vi "HFRR ADV v038 new software.vi"() -> ()   [LabVIEW 2025] (continued)
        n1338 = Not(x=w1631) -> (.not. x?=w1629:bool)
        n1339 = local write "Stroke"(w1629) -> ()
        n1340 = local write "Tab Control 2"(T6."Stroke" ("Tab Control 2")) -> ()
      }
    }
    n1341 = local write "tested by"(w1358) -> ()
    n1342 = case shown="True" w1354 {
      selector: w1354 -> [_ w1634]
      frame False {
      }
      frame True {
        n1343 = Not(x=w1634) -> (.not. x?=w1632:bool)
        n1344 = local write "Humidity 2"(w1632) -> ()
        n1345 = local write "Tab Control 2"(T6."Humidity" ("Tab Control 2")) -> ()
      }
    }
    n1346 = case shown="\"Calibration\"" "Main Dashboard Buttons" {
      tunnel: [T2."HOME" ("Main Tab") T2."Test Setup" ("Main Tab") T2."Acquire" ("Main Tab") T2."Adv Scar" ("Main Tab") T2."Adv Scar Report" ("Main Tab") T2."Compare Files" ("Main Tab") T2."Calibration" ("Main Tab") T2."About" ("Main Tab") T2."Advance" ("Main Tab")] -> w1337
      frame "Home", Default {
      }
      frame "Test Setup" {
      }
      frame "Dashboard" {
      }
      frame "Imaging" {
      }
      frame "Report" {
      }
      frame "Analysis" {
      }
      frame "Calibration" {
      }
      frame "About" {
      }
      frame "Advance" {
      }
    }
    n1347 = Wait (ms)(milliseconds to wait=u32 100) -> ()  [unwired: 1 out]
    n1348 = local read "Main Tab Display"() -> (w1357:T4)
    n1349 = local write "Main Tab"(w1337) -> ()
    n1350 = case shown="\"Dashboard 3\"" w1357 {
      frame "Dashboard 1", Default {
        n1351 = property on="Reset Graph" class="Bool (strict)"("Visible"=FALSE) -> ()  [unwired: 2 in, 2 out]
      }
      frame "Dashboard 2" {
        n1352 = property on="Reset Graph" class="Bool (strict)"("Visible"=TRUE) -> ()  [unwired: 2 in, 2 out]
      }
      frame "Dashboard 3" {
        n1353 = property on="Reset Graph" class="Bool (strict)"("Visible"=TRUE) -> ()  [unwired: 2 in, 2 out]
      }
    }
    n1354 = local read "SCAR MEASURMENT"() -> (w1345:enum32{"Auto Scar", "Manual Scar"})
    n1355 = local read "Humidity"() -> (w1359:bool)
    n1356 = local read "Cap Live Image"() -> (w1342:bool)
    n1357 = local read "Sample Temperature"() -> (w1352:bool)
    n1358 = local read "Air Temp vs Humidity"() -> (w1350:bool)
    n1359 = local read "Frequency"() -> (w1351:bool)
    n1360 = case shown="True" w1359 {
      frame False {
        n1361 = local write "Humidity On Command"(TRUE ("Humidity On Command")) -> ()
        n1362 = case shown="True" "Humidity Off Command" {
          selector: "Humidity Off Command" -> [_ w1647]
          frame False {
          }
          frame True {
            n1363 = stacked-sequence {
              frame #0 {
                n1364 = Wait (ms)(milliseconds to wait=u32 500) -> ()  [unwired: 1 out]
              }
              frame #1 {
                n1365 = local read "WriteHumidity"() -> (w1650:string[])
                n1366 = Insert Into Array(array=w1650, new element="R;1" ("new element/subarray")) -> (w1649:string[])  [unwired: 1 in]
                n1367 = local write "WriteHumidity"(w1649) -> ()
              }
              frame #2 {
                n1368 = Wait (ms)(milliseconds to wait=u32 500) -> ()  [unwired: 1 out]
              }
              frame #3 {
                n1369 = local read "WriteHumidity"() -> (w1653:string[])
                n1370 = local read "EVENT LOG"() -> (w1657:string)
                n1371 = call "Event Log.vi"("Content"="Humidity Control Off" ("string"), "EVENT LOG"=w1657) -> ("EVENT LOG"=w1658:string)  [unwired: 8 in, 1 out]
                n1372 = local write "EVENT LOG"(w1658) -> ()
                n1373 = Insert Into Array(array=w1653, new element="R;1" ("new element/subarray")) -> (w1654:string[])  [unwired: 1 in]
                n1374 = local write "WriteHumidity"(w1654) -> ()
              }
            }
            n1375 = Not(x=w1647) -> (.not. x?=w1646:bool)
            n1376 = local write "Humidity Off Command"(w1646) -> ()
          }
        }
      }
      frame True {
        n1377 = local write "Humidity Off Command"(TRUE ("Humidity Off Command")) -> ()
        n1378 = case shown="True" "Humidity On Command" {
          selector: "Humidity On Command" -> [_ w1662]
          frame False {
          }
          frame True {
            n1379 = stacked-sequence {
              frame #0 {
                n1380 = local read "Set Rh"() -> (w1668:dbl)
                n1381 = local read "WriteHumidity"() -> (w1664:string[])
                n1382 = Number To Fractional String(number=w1668, precision (6)=i16 2) -> (F-format string=w1669:string)  [unwired: 2 in]
                n1383 = Concatenate Strings("M;" ("new element/subarray"), w1669) -> (w1667:string)
                n1384 = Insert Into Array(array=w1664, new element=w1667) -> (w1663:string[])  [unwired: 1 in]
                n1385 = local write "WriteHumidity"(w1663) -> ()
              }
              frame #1 {
                n1386 = Wait (ms)(milliseconds to wait=u32 500) -> ()  [unwired: 1 out]
              }
              frame #2 {
                n1387 = local read "WriteHumidity"() -> (w1672:string[])
                n1388 = local read "Set Rh"() -> (w1676:dbl)
                n1389 = Number To Fractional String(number=w1676, precision (6)=i16 2) -> (F-format string=w1677:string)  [unwired: 2 in]
                n1390 = Concatenate Strings("M;" ("new element/subarray"), w1677) -> (w1675:string)
                n1391 = Insert Into Array(array=w1672, new element=w1675) -> (w1671:string[])  [unwired: 1 in]
                n1392 = local write "WriteHumidity"(w1671) -> ()
              }
              frame #3 {
                n1393 = Wait (ms)(milliseconds to wait=u32 500) -> ()  [unwired: 1 out]
              }
              frame #4 {
                (unwired) "% RH" ("string")
                (unwired) i16 2 ("precision (6)")
                (unwired) "M;" ("new element/subarray")
                n1394 = local read "Set Rh"() -> (w1686:dbl)
                n1395 = local read "WriteHumidity"() -> (w1679:string[])
                n1396 = Number To Fractional String(number=w1686, precision (6)=i16 2) -> (F-format string=w1683:string)  [unwired: 2 in]
                n1397 = Concatenate Strings("M;" ("new element/subarray"), w1683) -> (w1687:string)
                n1398 = Concatenate Strings("Humidity Set to : " ("string"), w1683, "% RH" ("string")) -> (w1681:string)
                n1399 = Insert Into Array(array=w1679, new element=w1687) -> (w1680:string[])  [unwired: 1 in]
                n1400 = disable-structure shown="Enabled" {
                  frame Enabled {
                    n1401 = local read "EVENT LOG"() -> (w1690:string)
                    n1402 = call "Event Log.vi"("Content"="Humidity Control On", "EVENT LOG"=w1690) -> ("EVENT LOG"=w1691:string)  [unwired: 8 in, 1 out]
                    n1403 = local write "EVENT LOG"(w1691) -> ()
                  }
                  frame Disabled {
                  }
                }
                n1404 = disable-structure shown="Enabled" {
                  disable-tunnel: w1681 -> [_ _]
                  frame Enabled {
                    n1405 = local read "EVENT LOG"() -> (w1693:string)
                    n1406 = call "Event Log.vi"("Content"="Humidity Control On", "EVENT LOG"=w1693) -> ("EVENT LOG"=w1694:string)  [unwired: 8 in, 1 out]
                    n1407 = local write "EVENT LOG"(w1694) -> ()
                  }
                  frame Disabled {
                  }
                }
                n1408 = local write "WriteHumidity"(w1680) -> ()
              }
            }
            n1409 = Not(x=w1662) -> (.not. x?=w1661:bool)
            n1410 = local write "Humidity On Command"(w1661) -> ()
          }
        }
      }
    }
    n1411 = Equal?(x=w1345, y=enum32{"Auto Scar", "Manual Scar"}."Auto Scar" ("SCAR MEASURMENT")) -> (x = y?=w1341:bool)
    n1412 = local read "TEST STANDARD"() -> (w1348:T3)
    n1413 = And(x=w1342, y=w1341) -> (x .and. y?=w1343:bool)
    n1414 = case shown="True" w1343 {
      selector: w1343 -> [_ w1446]
      tunnel: errorcluster {"status"=FALSE, "code"=0, "source"=""} ("error in (no error) 3") -> [_ w1447]
      frame False {
      }
      frame True {
        n1415 = stacked-sequence {
          tunnel: w1447 -> [_ _ _ _ _ _ _ w1495]
          tunnel: w1446 -> [_ _ _ _ _ w1476 _ _]
          frame #0 {
            n1416 = call "CAMERA LIVE FEED FGV.vi"("Enum - Menu"=CAMERA_LIVE_FEED_ENUM."CAMERA MINIMIZE") -> ()  [unwired: 9 in, 2 out]
          }
          frame #1 {
            n1417 = property on="Auto Scar Check  2" class="Clust (strict)"("Visible"=TRUE) -> ()  [unwired: 2 in, 2 out]
          }
          frame #2 {
            n1418 = String To Path(string="C:\\LAB-IQ\\Image Calibrate v01.dcf") -> (path=w1452:path)
            n1419 = Open/Create/Replace File ("Open File")(file path (use dialog)=w1452) -> (refnum out=w1453:refnum<file>)  [unwired: 5 in, 2 out]
            n1420 = for {
              N: 4 -> [_]
              tunnel: w1453 -> [w1459]
              i -> [w1455]
              n1421 = Read from Text File ("Read File")(file (use dialog)=w1459) -> (text=w1460:string)  [unwired: 3 in, 3 out]
              n1422 = String Subset(string=w1460, offset (0)=6, length (rest)=10 ("length (rest)")) -> (substring=w1456:string)
              n1423 = Fract/Exp String To Number(string=w1456) -> (number=w1454:dbl)  [unwired: 3 in, 1 out]
              n1424 = case shown="0" w1455 {
                tunnel: w1454 -> [w1461 w1462 _ w1463 _]
                frame 0 {
                  "5x Gain" <- w1461
                }
                frame 1 {
                  "10x Gain" <- w1462
                }
                frame 2 {
                }
                frame 3 {
                  "100x gain" <- w1463
                }
                frame 4, Default {
                }
              }
            }
          }
          frame #3 {
            n1425 = local read "FILE 3"() -> (w1469:string)
            n1426 = call <vilib>:"Trim Whitespace.vi"("string"="C:\\LAB-IQ\\images\\") -> ("trimmed string"=w1471:string)  [unwired: 1 in]
            n1427 = String To Path(string=w1471) -> (path=w1470:path)
            n1428 = Concatenate Strings(w1469, ".png" ("string")) -> (w1468:string)
            n1429 = Build Path(base path=w1470, name or relative path=w1468) -> (appended path=w1466:path)
            "Image path" <- w1466
            n1430 = Path To String(path=w1466) -> (string=w1465:string)
            n1431 = call "CAMERA LIVE FEED FGV.vi"("Enum - Menu"=CAMERA_LIVE_FEED_ENUM."CAMERA SAVE", "Image Path"=w1465) -> ()  [unwired: 8 in, 2 out]
          }
          frame #4 {
            n1432 = One Button Dialog(message="Image saved successfully") -> ()  [unwired: 1 in, 1 out]
          }
          frame #5 {
            n1433 = local read "TEST STANDARD"() -> (w1475:T3)
            n1434 = local read "Magnification len live scar"() -> (w1487:string)
            n1435 = Not(x=w1476) -> (.not. x?=w1477:bool)
            n1436 = local write "Cap Live Image"(w1477) -> ()
            n1437 = case shown="\"ISO 12156\"" w1475 {
              tunnel: ["ASTM D6079" "ISO 12156"] -> w1474
              frame "ASTM D6079", Default {
              }
              frame "ISO 12156" {
              }
            }
            n1438 = case shown="\"5x\", Default" w1487 {
              tunnel: [w1490 w1491] -> w1486
              frame "5x", Default {
                n1439 = local read "5x Gain"() -> (w1490:dbl)
              }
              frame "10x" {
                # "5x"
                n1440 = local read "10x Gain"() -> (w1491:dbl)
              }
            }
            n1441 = local read "Image path"() -> (w1485:path)
            n1442 = local read "FILE 3"() -> (w1478:string)
            n1443 = call "EDGE DETCTION.vi"("GAIN VALUE"=w1486, "Image Path"=w1485) -> ("error out"=w1484:errorcluster, "return value"=w1483:cluster{string, string, dbl, dbl, dbl})  [unwired: 8 in]
            n1444 = Bundle By Name(cluster=T26 {"File Name"="", "Test Method"="", "Operator"="", "Fuel Description"="", "Date and time"=""} ("Main Ref"), "File Name"=w1478, "Test Method"=w1474) -> (w1479:T26)
            n1445 = call "duf file read.vi"("error in (no error)"=w1484, "Main Ref"=w1479) -> ("error out"=w1482:errorcluster, "Main Ref 2"=w1480:T26)  [unwired: 8 in]
            n1446 = call "EDGE DETECTION REPORT.vi"("error in (no error)"=w1482, "return value 2"=w1483, "Main Ref"=w1480) -> ()  [unwired: 8 in, 1 out]
          }
          frame #6 {
            n1447 = property on="Auto Scar Check  2" class="Clust (strict)"("Visible"=FALSE) -> ()  [unwired: 2 in, 2 out]
          }
          frame #7 {
            n1448 = call "CAMERA LIVE FEED FGV.vi"("Enum - Menu"=CAMERA_LIVE_FEED_ENUM."CAMERA MINIMIZE", "error in (no error)"=w1495) -> ()  [unwired: 8 in, 2 out]
            n1449 = local write "Main Dashboard Buttons"(T1."Home" ("Main Dashboard Buttons")) -> ()
            n1450 = local write "Main Tab"(T2."HOME" ("Main Tab")) -> ()
          }
        }
      }
    }
    n1451 = local read "Heater Button"() -> (w1349:bool)
    n1452 = case shown="True" w1351 {
      selector: w1351 -> [_ w1625]
      frame False {
      }
      frame True {
        n1453 = Not(x=w1625) -> (.not. x?=w1623:bool)
        n1454 = local write "Frequency"(w1623) -> ()
        n1455 = local write "Tab Control 2"(T6."Frequency" ("Tab Control 2")) -> ()
      }
    }
    n1456 = case shown="True" w1350 {
      selector: w1350 -> [_ w1622]
      frame False {
      }
      frame True {
        n1457 = Not(x=w1622) -> (.not. x?=w1620:bool)
        n1458 = local write "Air Temp vs Humidity"(w1620) -> ()
        n1459 = local write "Tab Control 2"(T6."Air Temp vs Rh" ("Tab Control 2")) -> ()
      }
    }
    n1460 = case shown="True" w1352 {
      selector: w1352 -> [_ w1628]
      frame False {
      }
      frame True {
        n1461 = Not(x=w1628) -> (.not. x?=w1626:bool)
        n1462 = local write "Sample Temperature"(w1626) -> ()
        n1463 = local write "Tab Control 2"(T6."Sample Temperature" ("Tab Control 2")) -> ()
      }
    }
    n1464 = case shown="\"Custom\"" w1348 {
      frame "ASTM D6079", Default {
        w1601 = "ASTM D6079 TEST CONDITIONS" ("Standard 2")
        n1465 = local write "Standard 2"(w1601) -> ()
        n1466 = local write "Standard"(w1601) -> ()
      }
      frame "ISO 12156" {
        w1602 = "ISO 12156 TEST CONDITIONS" ("Standard 2")
        n1467 = local write "Standard 2"(w1602) -> ()
        n1468 = local write "Standard"(w1602) -> ()
      }
      frame "CEC F-096-A-06" {
        w1603 = "CEC F-096-A-06 TEST CONDITIONS" ("Standard 2")
        n1469 = local write "Standard 2"(w1603) -> ()
        n1470 = local write "Standard"(w1603) -> ()
      }
      frame "Custom" {
        w1604 = "CUSTOM TEST CONDITIONS" ("Standard 2")
        n1471 = local write "Standard 2"(w1604) -> ()
        n1472 = local write "Standard"(w1604) -> ()
      }
    }
    n1473 = case shown="True" w1349 {
      frame False {
        n1474 = local write "Temperature On Command"(TRUE ("Temperature On Command")) -> ()
        n1475 = case shown="True" "Temperature Off Command" {
          selector: "Temperature Off Command" -> [_ w1608]
          frame False {
          }
          frame True {
            n1476 = Not(x=w1608) -> (.not. x?=w1607:bool)
            n1477 = local read "EVENT LOG"() -> (w1611:string)
            n1478 = local write "Temperature Off Command"(w1607) -> ()
            n1479 = call "Event Log.vi"("Content"="Heater Off", "EVENT LOG"=w1611) -> ("EVENT LOG"=w1610:string)  [unwired: 8 in, 1 out]
            n1480 = local write "EVENT LOG"(w1610) -> ()
          }
        }
      }
      frame True {
        n1481 = local write "Temperature Off Command"(TRUE ("Temperature Off Command")) -> ()
        n1482 = case shown="True" "Temperature On Command" {
          selector: "Temperature On Command" -> [_ w1615]
          frame False {
          }
          frame True {
            n1483 = Not(x=w1615) -> (.not. x?=w1614:bool)
            n1484 = local write "Temperature On Command"(w1614) -> ()
            n1485 = disable-structure shown="Enabled" {
              disable-tunnel: "Heater On" -> [w1617 _]
              frame Enabled {
                n1486 = local read "EVENT LOG"() -> (w1618:string)
                n1487 = call "Event Log.vi"("Content"=w1617, "EVENT LOG"=w1618) -> ("EVENT LOG"=w1619:string)  [unwired: 8 in, 1 out]
                n1488 = local write "EVENT LOG"(w1619) -> ()
              }
              frame Disabled {
              }
            }
          }
        }
      }
    }
    n1489 = local read "Main Tab"() -> (w1340:T2)
    n1490 = case shown="\"About\"" w1340 {
      frame "HOME", Default {
        w1382 = T19."Enabled" ("Disabled")
        n1491 = local read "Service Password enable"() -> (w1384:bool)
        n1492 = property on="Imaging" class="Bool (strict)"("DisabledEnum"=w1382) -> ()  [unwired: 2 in, 2 out]
        n1493 = property on="Dashboard" class="Bool (strict)"("DisabledEnum"=w1382) -> ()  [unwired: 2 in, 2 out]
        n1494 = property on="Test Setup" class="Bool (strict)"("DisabledEnum"=w1382) -> ()  [unwired: 2 in, 2 out]
        n1495 = property on="Analysis" class="Bool (strict)"("DisabledEnum"=w1382) -> ()  [unwired: 2 in, 2 out]
        n1496 = property on="Home" class="Bool (strict)"("DisabledEnum"=w1382) -> ()  [unwired: 2 in, 2 out]
        n1497 = property on="Report" class="Bool (strict)"("DisabledEnum"=w1382) -> ()  [unwired: 2 in, 2 out]
        n1498 = property on="Main Dashboard Buttons" class="RadioBtnsControl (strict)"("DisabledEnum"=w1382) -> ()  [unwired: 2 in, 2 out]
        n1499 = property on="Calibration" class="Bool (strict)"("DisabledEnum"=w1382) -> ()  [unwired: 2 in, 2 out]
        n1500 = case shown="True" w1384 {
          tunnel: [T19."Disabled" ("Disabled") T19."Enabled" ("Disabled")] -> w1383
          frame False {
          }
          frame True {
          }
        }
        n1501 = property on="About" class="Bool (strict)"("DisabledEnum"=w1383) -> ()  [unwired: 2 in, 2 out]
      }
      frame "Test Setup" {
        w1389 = T19."Enabled" ("Disabled")
        n1502 = local read "Service Password enable"() -> (w1388:bool)
        n1503 = property on="Dashboard" class="Bool (strict)"("DisabledEnum"=T19."Disabled" ("Disabled")) -> ()  [unwired: 2 in, 2 out]
        n1504 = property on="Imaging" class="Bool (strict)"("DisabledEnum"=w1389) -> ()  [unwired: 2 in, 2 out]
        n1505 = property on="Analysis" class="Bool (strict)"("DisabledEnum"=w1389) -> ()  [unwired: 2 in, 2 out]
        n1506 = property on="Home" class="Bool (strict)"("DisabledEnum"=w1389) -> ()  [unwired: 2 in, 2 out]
        n1507 = property on="Report" class="Bool (strict)"("DisabledEnum"=w1389) -> ()  [unwired: 2 in, 2 out]
        n1508 = property on="Test Setup" class="Bool (strict)"("DisabledEnum"=w1389) -> ()  [unwired: 2 in, 2 out]
        n1509 = case shown="True" w1388 {
          tunnel: [T19."Disabled" ("Disabled") T19."Enabled" ("Disabled")] -> w1387
          frame False {
          }
          frame True {
          }
        }
        n1510 = property on="About" class="Bool (strict)"("DisabledEnum"=w1387) -> ()  [unwired: 2 in, 2 out]
      }
      frame "Adv Scar" {
        w1396 = T19."Enabled" ("Disabled")
        n1511 = property on="Dashboard" class="Bool (strict)"("DisabledEnum"=T19."Disabled" ("Disabled")) -> ()  [unwired: 2 in, 2 out]
        n1512 = property on="Imaging" class="Bool (strict)"("DisabledEnum"=w1396) -> ()  [unwired: 2 in, 2 out]
        n1513 = property on="Analysis" class="Bool (strict)"("DisabledEnum"=w1396) -> ()  [unwired: 2 in, 2 out]
        n1514 = property on="Home" class="Bool (strict)"("DisabledEnum"=w1396) -> ()  [unwired: 2 in, 2 out]
        n1515 = property on="Report" class="Bool (strict)"("DisabledEnum"=w1396) -> ()  [unwired: 2 in, 2 out]
        n1516 = property on="Test Setup" class="Bool (strict)"("DisabledEnum"=w1396) -> ()  [unwired: 2 in, 2 out]
        n1517 = local read "Service Password enable"() -> (w1394:bool)
        n1518 = case shown="True" w1394 {
          tunnel: [T19."Disabled" ("Disabled") T19."Enabled" ("Disabled")] -> w1393
          frame False {
          }
          frame True {
          }
        }
        n1519 = property on="About" class="Bool (strict)"("DisabledEnum"=w1393) -> ()  [unwired: 2 in, 2 out]
      }
      frame "Calibration" {
        w1399 = T19."Enabled" ("Disabled")
        n1520 = property on="Dashboard" class="Bool (strict)"("DisabledEnum"=T19."Disabled" ("Disabled")) -> ()  [unwired: 2 in, 2 out]
        n1521 = property on="Imaging" class="Bool (strict)"("DisabledEnum"=w1399) -> ()  [unwired: 2 in, 2 out]
        n1522 = property on="Analysis" class="Bool (strict)"("DisabledEnum"=w1399) -> ()  [unwired: 2 in, 2 out]
        n1523 = property on="Home" class="Bool (strict)"("DisabledEnum"=w1399) -> ()  [unwired: 2 in, 2 out]
        n1524 = property on="Report" class="Bool (strict)"("DisabledEnum"=w1399) -> ()  [unwired: 2 in, 2 out]
        n1525 = property on="Test Setup" class="Bool (strict)"("DisabledEnum"=w1399) -> ()  [unwired: 2 in, 2 out]
        n1526 = local read "Service Password enable"() -> (w1401:bool)
        n1527 = property on="Calibration" class="Bool (strict)"("DisabledEnum"=w1399) -> ()  [unwired: 2 in, 2 out]
        n1528 = case shown="True" w1401 {
          tunnel: [T19."Disabled" ("Disabled") T19."Enabled" ("Disabled")] -> w1400
          frame False {
          }
          frame True {
          }
        }
        n1529 = property on="About" class="Bool (strict)"("DisabledEnum"=w1400) -> ()  [unwired: 2 in, 2 out]
      }
      frame "Adv Scar Report" {
        w1407 = T19."Enabled" ("Disabled")
        n1530 = property on="Dashboard" class="Bool (strict)"("DisabledEnum"=T19."Disabled" ("Disabled")) -> ()  [unwired: 2 in, 2 out]
        n1531 = property on="Imaging" class="Bool (strict)"("DisabledEnum"=w1407) -> ()  [unwired: 2 in, 2 out]
        n1532 = property on="Analysis" class="Bool (strict)"("DisabledEnum"=w1407) -> ()  [unwired: 2 in, 2 out]
        n1533 = property on="Home" class="Bool (strict)"("DisabledEnum"=w1407) -> ()  [unwired: 2 in, 2 out]
        n1534 = property on="Report" class="Bool (strict)"("DisabledEnum"=w1407) -> ()  [unwired: 2 in, 2 out]
        n1535 = property on="Test Setup" class="Bool (strict)"("DisabledEnum"=w1407) -> ()  [unwired: 2 in, 2 out]
        n1536 = local read "Service Password enable"() -> (w1406:bool)
        n1537 = case shown="True" w1406 {
          tunnel: [T19."Disabled" ("Disabled") T19."Enabled" ("Disabled")] -> w1405
          frame False {
          }
          frame True {
          }
        }
        n1538 = property on="About" class="Bool (strict)"("DisabledEnum"=w1405) -> ()  [unwired: 2 in, 2 out]
      }
      frame "Compare Files" {
        w1413 = T19."Enabled" ("Disabled")
        n1539 = local read "Service Password enable"() -> (w1412:bool)
        n1540 = property on="Dashboard" class="Bool (strict)"("DisabledEnum"=T19."Disabled" ("Disabled")) -> ()  [unwired: 2 in, 2 out]
        n1541 = property on="Imaging" class="Bool (strict)"("DisabledEnum"=w1413) -> ()  [unwired: 2 in, 2 out]
        n1542 = property on="Analysis" class="Bool (strict)"("DisabledEnum"=w1413) -> ()  [unwired: 2 in, 2 out]
        n1543 = property on="Home" class="Bool (strict)"("DisabledEnum"=w1413) -> ()  [unwired: 2 in, 2 out]
        n1544 = property on="Report" class="Bool (strict)"("DisabledEnum"=w1413) -> ()  [unwired: 2 in, 2 out]
        n1545 = property on="Test Setup" class="Bool (strict)"("DisabledEnum"=w1413) -> ()  [unwired: 2 in, 2 out]
        n1546 = case shown="True" w1412 {
          tunnel: [T19."Disabled" ("Disabled") T19."Enabled" ("Disabled")] -> w1411
          frame False {
          }
          frame True {
          }
        }
        n1547 = property on="About" class="Bool (strict)"("DisabledEnum"=w1411) -> ()  [unwired: 2 in, 2 out]
      }
      frame "Acquire" {
        n1548 = local read "Service Password enable"() -> (w1418:bool)
        n1549 = property on="Test Setup" class="Bool (strict)"("DisabledEnum"=T19."Disabled" ("Disabled")) -> ()  [unwired: 2 in, 2 out]
        n1550 = local read "Auto Start Test"() -> (w1420:bool)
        n1551 = local read "RUN"() -> (w1422:bool)
        n1552 = case shown="True" w1418 {
          tunnel: [T19."Disabled" ("Disabled") T19."Enabled" ("Disabled")] -> w1419
          frame False {
          }
          frame True {
          }
        }
        n1553 = Or(x=w1422, y=w1420) -> (x .or. y?=w1421:bool)
        n1554 = case shown="True" w1421 {
          tunnel: [T19."Enabled" ("Disabled") T19."Disabled" ("Disabled")] -> w1417
          frame False {
          }
          frame True {
          }
        }
        n1555 = property on="About" class="Bool (strict)"("DisabledEnum"=w1419) -> ()  [unwired: 2 in, 2 out]
        n1556 = property on="Imaging" class="Bool (strict)"("DisabledEnum"=w1417) -> ()  [unwired: 2 in, 2 out]
        n1557 = property on="Dashboard" class="Bool (strict)"("DisabledEnum"=w1417) -> ()  [unwired: 2 in, 2 out]
        n1558 = property on="Analysis" class="Bool (strict)"("DisabledEnum"=w1417) -> ()  [unwired: 2 in, 2 out]
        n1559 = property on="Home" class="Bool (strict)"("DisabledEnum"=w1417) -> ()  [unwired: 2 in, 2 out]
        n1560 = property on="Report" class="Bool (strict)"("DisabledEnum"=w1417) -> ()  [unwired: 2 in, 2 out]
        n1561 = property on="Calibration" class="Bool (strict)"("DisabledEnum"=w1417) -> ()  [unwired: 2 in, 2 out]
      }
      frame "About" {
        n1562 = local read "FILE"() -> (w1436:string)
        n1563 = local read "TEST FILE NAM,E SAVED"() -> (w1429:bool)
        n1564 = call <vilib>:"Trim Whitespace.vi"("string"=w1436) -> ("trimmed string"=w1435:string)  [unwired: 1 in]
        n1565 = local read "Auto Start Test"() -> (w1439:bool)
        n1566 = String Length(string=w1435) -> (length=w1434:i32)
        n1567 = Greater?(x=w1434, y=1) -> (0:w1431:bool)
        n1568 = And(x=w1431, y=w1429) -> (x .and. y?=w1430:bool)
        n1569 = local read "RUN"() -> (w1441:bool)
        n1570 = case shown="True" w1430 {
          tunnel: [T19."Disabled" ("Disabled") T19."Enabled" ("Disabled")] -> w1432
          frame False {
          }
          frame True {
          }
        }
        n1571 = Or(x=w1441, y=w1439) -> (x .or. y?=w1440:bool)
        n1572 = property on="About" class="Bool (strict)"("DisabledEnum"=T19."Enabled" ("Disabled")) -> ()  [unwired: 2 in, 2 out]
        n1573 = case shown="False" w1440 {
          tunnel: [T19."Enabled" ("Disabled") T19."Disabled" ("Disabled")] -> w1438
          frame False {
          }
          frame True {
          }
        }
        n1574 = property on="Dashboard" class="Bool (strict)"("DisabledEnum"=w1432) -> ()  [unwired: 2 in, 2 out]
        n1575 = property on="Test Setup" class="Bool (strict)"("DisabledEnum"=T19."Disabled" ("Disabled")) -> ()  [unwired: 2 in, 2 out]
        n1576 = property on="Imaging" class="Bool (strict)"("DisabledEnum"=w1438) -> ()  [unwired: 2 in, 2 out]
        n1577 = property on="Analysis" class="Bool (strict)"("DisabledEnum"=w1438) -> ()  [unwired: 2 in, 2 out]
        n1578 = property on="Home" class="Bool (strict)"("DisabledEnum"=w1438) -> ()  [unwired: 2 in, 2 out]
        n1579 = property on="Report" class="Bool (strict)"("DisabledEnum"=w1438) -> ()  [unwired: 2 in, 2 out]
      }
    }
    n1580 = local read "Quit"() -> (w1366:bool)
    "Single" <- "Single - Graph"
  }
  n1581 = disable-structure shown="Disabled" {
    disable-tunnel: [w1719 _] -> w42
    disable-tunnel: _ -> [w1718 _]
    frame Disabled {
      n1582 = while {
        tunnel: w1718 -> [_]
        tunnel: [w1720] -> w1719
        tunnel: [w1721] -> _
        i -> [w1721]
        stop <- w1720 stop-if-true
        w1737 = u16 10 items=["1.0"=10, "1.5"=15, "2.0"=20] ("stop bits (10: 1 bit)")
        n1583 = Wait (ms)(milliseconds to wait=u32 10) -> ()  [unwired: 1 out]
        n1584 = call-poly "VISA Configure Serial Port"("VISA resource name"=refnum<visa-resource-name> "ASRL1::INSTR" ("COM PORT"), "timeout (10sec)"=u32 10, "baud rate (9600)"=u32 57600, "data bits (8)"=u16 8, "stop bits (10: 1 bit)"=w1737) -> ("VISA resource name out"=w1723:refnum<visa-resource-name>, "error out"=w1732:errorcluster)  [unwired: 9 in]
        n1585 = VISA Read(VISA resource name=w1723, byte count=u32 2 ("byte count (0)")) -> (read buffer=w1731:string)  [unwired: 1 in, 3 out]
        n1586 = String Subset(string=w1731, offset (0)=0, length (rest)=2 ("length (rest)")) -> (substring=w1730:string)
        n1587 = Match Pattern(string=w1730, regular expression="<>") -> (offset past match=w1727:i32)  [unwired: 1 in, 3 out]
        n1588 = Greater Or Equal?(x=w1727, y=0) -> (x >= y?=w1722:bool)
        n1589 = case shown="True" w1722 {
          tunnel: w1723 -> [_ w1741]
          tunnel: w1732 -> [_ w1740]
          frame False {
          }
          frame True {
            n1590 = VISA Read(VISA resource name=w1741, byte count=u32 32 ("byte count (0)"), error in (no error)=w1740) -> (read buffer=w1739:string)  [unwired: 3 out]
            n1591 = String Subset(string=w1739, offset (0)=0, length (rest)=8 ("length (rest)")) -> (substring=w1743:string)
            n1592 = String Subset(string=w1739, offset (0)=8, length (rest)=8 ("length (rest)")) -> (substring=w1744:string)
            n1593 = Decimal String To Number(string=w1744) -> (number=w1751:i32)  [unwired: 2 in, 1 out]
            n1594 = Decimal String To Number(string=w1743) -> (number=w1747:i32)  [unwired: 2 in, 1 out]
            n1595 = Divide(x=w1751, y=10000) -> ()  [unwired: 1 out]
            n1596 = Divide(x=w1747, y=1000000) -> ()  [unwired: 1 out]
          }
        }
        n1597 = local read "Quit"() -> (w1720:bool)
      }
    }
    frame Enabled {
    }
  }
  n1598 = Tick Count (ms)() -> (millisecond timer value=w4:u32)
  n1599 = while {
    shift-right: [w1797] -> _
    shift-left: w6 -> [w1801]
    shift-right: [w1796] -> _
    shift-left: w5 -> [w1800]
    shift-right: [w1795] -> _
    shift-left: w6 -> [w1799]
    shift-right: [w1794] -> _
    shift-left: w5 -> [w1798]
    shift-right: [w1792] -> _
    shift-left: w4 -> [w1793]
    shift-right: [w1789] -> _
    shift-left: w3 -> [w1790]
    shift-right: [w1788] -> _
    shift-left: w3 -> [w1791]
    shift-right: [w1781] -> _
    shift-left: w3 -> [w1787]
    shift-right: [w1780] -> _
    shift-left: w3 -> [w1786]
    shift-right: [w1779] -> _
    shift-left: w3 -> [w1785]
    shift-right: [w1778] -> _
    shift-left: w3 -> [w1784]
    shift-right: [w1777] -> _
    shift-left: w3 -> [w1783]
    shift-right: [w1776] -> _
    shift-left: w3 -> [w1782]
    shift-right: [w1775] -> _
    shift-left: w3 -> [w1769]
    shift-right: [w1774] -> _
    shift-left: w3 -> [w1768]
    shift-right: [w1773] -> _
    shift-left: w3 -> [w1767]
    shift-right: [w1772] -> _
    shift-left: w3 -> [w1766]
    shift-right: [w1771] -> _
    shift-left: w3 -> [w1765]
    shift-right: [w1770] -> _
    shift-left: w3 -> [w1764]
    shift-right: [w1755] -> _
    shift-left: w3 -> [w1758]
    shift-right: [w1754] -> _
    shift-left: w3 -> [w1757]
    shift-right: [w1753] -> _
    shift-left: w3 -> [w1756]
    stop <- w1803 stop-if-true
    n1600 = local read "Read UNO"() -> (w1762:string)
    n1601 = local read "Error  2"() -> (w1802:errorcluster)
    n1602 = String Length(string=w1762) -> (length=w1761:i32)
    n1603 = call <vilib>:"Trim Whitespace.vi"("string"=w1762) -> ("trimmed string"=w1763:string)  [unwired: 1 in]
    n1604 = Greater Or Equal?(x=w1761, y=23) -> (x >= y?=w1759:bool)
    n1605 = case shown="No Error" w1802 {
      tunnel: w1801 -> [w1849 w1945]
      tunnel: w1800 -> [w1848 w1944]
      tunnel: w1799 -> [w1847 w1943]
      tunnel: w1798 -> [w1846 w1942]
      tunnel: [w1845 w1945] -> w1797
      tunnel: [w1844 w1944] -> w1796
      tunnel: [w1843 w1943] -> w1795
      tunnel: [w1842 w1942] -> w1794
      tunnel: w1793 -> [w1841 w1941]
      tunnel: [w1840 w1941] -> w1792
      tunnel: w1790 -> [w1839 w1940]
      tunnel: w1791 -> [w1838 w1939]
      tunnel: [w1837 w1940] -> w1789
      tunnel: [w1836 w1939] -> w1788
      tunnel: w1787 -> [w1835 w1938]
      tunnel: w1786 -> [w1834 w1937]
      tunnel: w1785 -> [w1833 w1936]
      tunnel: w1784 -> [w1832 w1935]
      tunnel: w1783 -> [w1831 w1934]
      tunnel: w1782 -> [w1830 w1933]
      tunnel: [w1829 w1938] -> w1781
      tunnel: [w1828 w1937] -> w1780
      tunnel: [w1827 w1936] -> w1779
      tunnel: [w1826 w1935] -> w1778
      tunnel: [w1825 w1934] -> w1777
      tunnel: [w1824 w1933] -> w1776
      tunnel: w1769 -> [w1823 w1932]
      tunnel: [w1822 w1932] -> w1775
      tunnel: [w1821 w1928] -> w1774
      tunnel: [w1820 w1927] -> w1773
      tunnel: [w1819 w1931] -> w1772
      tunnel: [w1818 w1930] -> w1771
      tunnel: [w1817 w1929] -> w1770
      tunnel: w1768 -> [w1816 w1931]
      tunnel: w1767 -> [w1815 w1930]
      tunnel: w1766 -> [w1814 w1929]
      tunnel: w1765 -> [w1813 w1928]
      tunnel: w1764 -> [w1812 w1927]
      tunnel: w1763 -> [w1811 _]
      tunnel: w1759 -> [w1810 _]
      tunnel: w1758 -> [w1809 w1926]
      tunnel: w1757 -> [w1808 w1925]
      tunnel: w1756 -> [w1807 w1924]
      tunnel: [w1806 w1926] -> w1755
      tunnel: [w1805 w1925] -> w1754
      tunnel: [w1804 w1924] -> w1753
      frame No Error {
        n1606 = case shown="True" w1810 {
          tunnel: w1849 -> [w1865 w1917]
          tunnel: w1848 -> [w1864 w1916]
          tunnel: w1847 -> [w1863 w1915]
          tunnel: w1846 -> [w1862 w1914]
          tunnel: [w1865 w1913] -> w1845
          tunnel: [w1864 w1912] -> w1844
          tunnel: [w1863 w1911] -> w1843
          tunnel: [w1862 w1910] -> w1842
          tunnel: w1841 -> [w1861 w1908]
          tunnel: [w1861 w1907] -> w1840
          tunnel: w1839 -> [w1860 w1906]
          tunnel: w1838 -> [w1859 w1905]
          tunnel: [w1860 w1904] -> w1837
          tunnel: [w1859 w1903] -> w1836
          tunnel: w1835 -> [w1858 w1902]
          tunnel: w1834 -> [w1857 w1901]
          tunnel: w1833 -> [w1856 w1900]
          tunnel: w1832 -> [w1855 w1899]
          tunnel: w1831 -> [w1854 w1898]
          tunnel: w1830 -> [w1853 w1897]
          tunnel: [w1858 w1896] -> w1829
          tunnel: [w1857 w1895] -> w1828
          tunnel: [w1856 w1894] -> w1827
          tunnel: [w1855 w1893] -> w1826
          tunnel: [w1854 w1892] -> w1825
          tunnel: [w1853 w1891] -> w1824
          tunnel: w1823 -> [w1871 w1890]
          tunnel: [w1871 w1889] -> w1822
          tunnel: [w1868 w1888] -> w1821
          tunnel: [w1867 w1887] -> w1820
          tunnel: [w1870 w1886] -> w1819
          tunnel: [w1866 w1885] -> w1818
          tunnel: [w1869 w1884] -> w1817
          tunnel: w1816 -> [w1870 w1883]
          tunnel: w1815 -> [w1869 w1882]
          tunnel: w1814 -> [w1868 w1881]
          tunnel: w1813 -> [w1867 w1880]
          tunnel: w1812 -> [w1866 w1879]
          tunnel: w1811 -> [_ w1878]
          tunnel: w1809 -> [w1852 w1877]
          tunnel: w1808 -> [w1851 w1876]
          tunnel: w1807 -> [w1850 w1875]
          tunnel: [w1852 w1874] -> w1806
          tunnel: [w1851 w1873] -> w1805
          tunnel: [w1850 w1872] -> w1804
          frame False {
          }
          frame True {
            n1607 = Tick Count (ms)() -> (millisecond timer value=w1909:u32)
            n1608 = String To Byte Array(string=w1878) -> (unsigned byte array=w1922:u8[])
            n1609 = Array Size(array=w1922) -> (size(s)=w1921:i32)
            n1610 = formula code="// --- INTERNAL VARIABLE DECLARATIONS ---\nint i = 0;\nint k = 0;\nint start_idx = -1;\nint end_idx = -1;\nint phase = 0;\nint sign0 = 1;\nint sign1 = 1;\nint ch0_val = 0;   \nint ch1_val = 0;   \nfloat ch0_raw = 0.0;\nfloat ch1_raw = 0.0;\nfloat temp0 = 0.0;\nfloat temp1 = 0.0;\nfloat ch0_clean = 0.0;\nfloat ch1_clean = 0.0;\n\nint valid_samples = 0; // FIX: Track if we actually parsed new data this window\nfloat max_allowed_bits = 8388607.0; // FIX: Change this to match your ADC max value\n\n// Temporal intermediate variables for calculation smoothing\nfloat raw_p2p_v = 0.0;\nfloat raw_friction = 0.0;\nfloat raw_cof = 0.0;\n\n// Temporal intermediate variables for Piezo voltage translations\nfloat piezo_min_v = 0.0;\nfloat piezo_max_v = 0.0;\n\n// Initialize output variables to current shift register states right away\nout_LVDT_Min_V = in_LVDT_Min_V;\nout_LVDT_Max_V = in_LVDT_Max_V;\nout_LVDT_P2P_V = in_LVDT_P2P_V;\nout_Piezo_P2P = in_Piezo_P2P;\nout_Friction_N = in_Friction_N;\nout_COF = in_COF;\nwindow_ready = 0;\n\n// --- STEP 1: PARSE EVERY STRING IN THE BYTE ARRAY ---\nif (array_size > 2) {\n    for (i = 0; i < array_size - 1; i++) {\n        if (raw_bytes[i] == 42) { // '*' character detected\n            start_idx = i;\n        }\n        \n        // Match standard delimiter sequence \";&\" or end window character\n        if (raw_bytes[i] == 59 && raw_bytes[i+1] == 38 && start_idx != -1) { \n            end_idx = i;\n            ch0_val = 0;\n            ch1_val = 0;\n            sign0 = 1;\n            sign1 = 1;\n            phase = 0; \n\n            for (k = start_idx + 1; k < end_idx; k++) {\n                if (raw_bytes[k] == 45) { // '-' sign\n                    if (phase == 0) sign0 = -1;\n                    else sign1 = -1;\n                }\n                else if (raw_bytes[k] == 43) { // '+' sign\n                    if (phase == 0) sign0 = 1;\n                    else sign1 = 1;\n                }\n                else if (raw_bytes[k] == 59) { // ';' delimiter\n                    phase = 1; \n                }\n                else if (raw_bytes[k] >= 48 && raw_bytes[k] <= 57) { // Numeric ASCII digits\n                    if (phase == 0) {\n                        ch0_val = (ch0_val * 10) + (raw_bytes[k] - 48);\n                    } else {\n                        ch1_val = (ch1_val * 10) + (raw_bytes[k] - 48);\n                    }\n                }\n            }\n\n            // Implicit type conversion\n            ch0_raw = ch0_val * sign0 * 1.0;\n            ch1_raw = ch1_val * sign1 * 1.0;\n\n            // FIX: Sanity check / Hard-clamping to catch sudden massive ASCII noise spikes\n            if (ch0_raw > max_allowed_bits)  ch0_raw = max_allowed_bits;\n            if (ch0_raw < -max_allowed_bits) ch0_raw = -max_allowed_bits;\n            if (ch1_raw > max_allowed_bits)  ch1_raw = max_allowed_bits;\n            if (ch1_raw < -max_allowed_bits) ch1_raw = -max_allowed_bits;\n\n            // --- STEP 2: 3-SAMPLE MEDIAN FILTER ---\n            m0_2 = m0_1; m0_1 = m0_0; m0_0 = ch0_raw;\n            float s0_0 = m0_0; float s0_1 = m0_1; float s0_2 = m0_2;\n            if (s0_0 > s0_1) { temp0 = s0_0; s0_0 = s0_1; s0_1 = temp0; }\n            if (s0_1 > s0_2) { temp0 = s0_1; s0_1 = s0_2; s0_2 = temp0; }\n            if (s0_0 > s0_1) { temp0 = s0_0; s0_0 = s0_1; s0_1 = temp0; }\n            ch0_clean = s0_1;\n\n            m1_2 = m1_1; m1_1 = m1_0; m1_0 = ch1_raw;\n            float s1_0 = m1_0; float s1_1 = m1_1; float s1_2 = m1_2;\n            if (s1_0 > s1_1) { temp1 = s1_0; s1_0 = s1_1; s1_1 = temp1; }\n            if (s1_1 > s1_2) { temp1 = s1_1; s1_1 = s1_2; s1_2 = temp1; }\n            if (s1_0 > s1_1) { temp1 = s1_0; s1_0 = s1_1; s1_1 = temp1; }\n            ch1_clean = s1_1;\n\n            // --- STEP 3: EXPONENTIAL FILTER (STREAM LEVEL) ---\n            if (ch0_filt == 0.0) ch0_filt = ch0_clean;\n            if (ch1_filt == 0.0) ch1_filt = ch1_clean;\n\n            ch0_filt = ch0_filt + (ch0_clean - ch0_filt) * 0.125;\n            ch1_filt = ch1_filt + (ch1_clean - ch1_filt) * 0.125;\n\n            // --- STEP 4: MIN/MAX WINDOW CONTINUOUS ACCUMULATION ---\n            if (ch0_filt > max_ch0) max_ch0 = ch0_filt;\n            if (ch0_filt < min_ch0) min_ch0 = ch0_filt;\n            if (ch1_filt > max_ch1) max_ch1 = ch1_filt;\n            if (ch1_filt < min_ch1) min_ch1 = ch1_filt;\n\n            valid_samples++; // FIX: Successfully parsed and accumulated a clean point\n            start_idx = -1; \n        }\n    }\n}\n\n// --- STEP 5: WINDOW EVALUATION ENGINE ---\n// FIX: Condition updated to verify that valid samples exist for both channels\nif (((current_time_ms - start_time_ms) >= 50) && (valid_samples > 0) && (min_ch0 < 9000000.0) && (min_ch1 < 9000000.0)) {\n    window_ready = 1;\n\n    // Linear Bit-to-Voltage Transformations (LVDT - Channel 0)\n    out_LVDT_Min_V = (min_ch0 * VREF) / 8388607.0;\n    out_LVDT_Max_V = (max_ch0 * VREF) / 8388607.0;\n    raw_p2p_v = out_LVDT_Max_V - out_LVDT_Min_V;\n\n    // Linear Bit-to-Voltage Transformations (Piezo - Channel 1)\n    piezo_min_v = (min_ch1 * VREF) / 8388607.0;\n    piezo_max_v = (max_ch1 * VREF) / 8388607.0;\n    \n    // Assign Peak-to-Peak Voltage directly to output indicator (Matches Python logic)\n    out_Piezo_P2P = piezo_max_v - piezo_min_v;\n    \n    // Force scaling calculations using Voltage delta * Newtons/Volt Factor\n    raw_friction = out_Piezo_P2P * PIEZO_CAL_FACTOR + 0.44528;\n    raw_cof = raw_friction / NORMAL_FORCE;\n\n    // --- STEP 6: OUTPUT METRIC SMOOTHING (Low-Pass Filter Alpha = 0.05) ---\n    // Seed initial historical metrics if first loop iteration\n    if (hist_LVDT_P2P == 0.0) hist_LVDT_P2P = raw_p2p_v;\n    if (hist_Friction == 0.0) hist_Friction = raw_friction;\n    if (hist_COF == 0.0)      hist_COF = raw_cof;\n\n    // Apply exponential output dampening\n    hist_LVDT_P2P = hist_LVDT_P2P + (raw_p2p_v - hist_LVDT_P2P) * 0.05;\n    hist_Friction = hist_Friction + (raw_friction - hist_Friction) * 0.05; // Note: Can drop to 0.02 for more aggressive damping\n    hist_COF      = hist_COF + (raw_cof - hist_COF) * 0.05;\n\n    // Direct smoothed parameters out to UI Indicators\n    out_LVDT_P2P_V = hist_LVDT_P2P;\n    out_Friction_N = hist_Friction;\n    out_COF        = hist_COF;\n\n    // Reset tracking targets to extreme boundaries safely\n    min_ch0 = 9999999.0;\n    max_ch0 = -9999999.0;\n    min_ch1 = 9999999.0;\n    max_ch1 = -9999999.0;\n\n    valid_samples = 0; // FIX: Reset counter for next time frame\n    start_time_ms = current_time_ms;\n}"("raw_bytes"=w1922, "array_size"=w1921, "VREF"="VREF", "PIEZO_CAL_FACTOR"="PIEZO_CAL_FACTOR", "NORMAL_FORCE"="NORMAL_FORCE", "min_ch0"=w1917, "max_ch0"=w1916, "min_ch1"=w1915, "max_ch1"=w1914, "current_time_ms"=w1909, "start_time_ms"=w1908, "ch0_filt"=w1906, "ch1_filt"=w1905, "m0_0"=w1902, "m0_1"=w1901, "m0_2"=w1900, "m1_0"=w1899, "m1_1"=w1898, "m1_2"=w1897, "in_LVDT_Min_V"=w1890, "in_LVDT_Max_V"=w1883, "in_LVDT_P2P_V"=w1882, "in_Piezo_P2P"=w1881, "in_Friction_N"=w1880, "in_COF"=w1879, "hist_LVDT_P2P"=w1877, "hist_Friction"=w1876, "hist_COF"=w1875) -> ("window_ready"=→"Valid_data":dbl, "out_LVDT_Min_V"=w1889:dbl, "out_LVDT_Max_V"=w1888:dbl, "out_LVDT_P2P_V"=w1887:dbl, "out_Piezo_P2P"=w1886:dbl, "out_Friction_N"=w1885:dbl, "out_COF"=w1884:dbl, "min_ch0"=w1913:dbl, "max_ch0"=w1912:dbl, "min_ch1"=w1911:dbl, "max_ch1"=w1910:dbl, "start_time_ms"=w1907:u32, "ch0_filt"=w1904:dbl, "ch1_filt"=w1903:dbl, "m0_0"=w1896:dbl, "m0_1"=w1895:dbl, "m0_2"=w1894:dbl, "m1_0"=w1893:dbl, "m1_1"=w1892:dbl, "m1_2"=w1891:dbl, "hist_LVDT_P2P"=w1874:dbl, "hist_Friction"=w1873:dbl, "hist_COF"=w1872:dbl)
            "LVDT MIN" <- w1889
            "LVDT MAX" <- w1888
            "LVDT Peak" <- w1887
            "pizo raw" <- w1886
            "cof" <- w1884
            "Frictioin Force Raw" <- w1885
          }
        }
      }
      frame Error {
      }
    }
    n1611 = local read "Quit"() -> (w1803:bool)
  }
  n1612 = disable-structure shown="Disabled" {
    disable-tunnel: errorcluster {"status"=TRUE, "code"=0, "source"="Init"} ("error IO") -> [w1948 _]
    disable-tunnel: [w1946 _] -> w45
    frame Disabled {
      n1613 = while {
        shift-right: [w1964] -> w1950
        shift-left: _ -> [w1955]
        shift-right: [w1963] -> w1949
        shift-left: w1948 -> [w1957]
        tunnel: [w1952] -> w1946
        tunnel: [w1962] -> _
        i -> [w1962]
        stop <- w1952 stop-if-true
        n1614 = local read "Port 1a"() -> (w1958:bool)
        n1615 = local read "Port 3"() -> (w1959:bool)
        n1616 = local read "Com Port 1"() -> (w1956:refnum<visa-resource-name>)
        n1617 = Or(x=w1959, y=w1958) -> (x .or. y?=w1961:bool)
        n1618 = Unbundle(w1957) -> ("status"=→"Port 3":bool)  [unwired: 2 out]
        n1619 = Not Equal?(x=w1956, y=w1955) -> (x != y?=w1953:bool)
        n1620 = case shown="True" w1961 {
          frame False {
            w1967 = TRUE ("Visible")
            n1621 = property on="Port 1a" class="Bool (strict)"("Visible"=w1967) -> ()  [unwired: 2 in, 2 out]
            n1622 = property on="Port 3" class="Bool (strict)"("Visible"=w1967) -> ()  [unwired: 2 in, 2 out]
          }
          frame True {
            w1968 = TRUE ("Visible")
            n1623 = property on="Port 1a" class="Bool (strict)"("Visible"=w1968) -> ()  [unwired: 2 in, 2 out]
            n1624 = property on="Port 3" class="Bool (strict)"("Visible"=w1968) -> ()  [unwired: 2 in, 2 out]
          }
        }
        n1625 = Wait (ms)(milliseconds to wait=u32 40) -> ()  [unwired: 1 out]
        n1626 = case shown="True" w1953 {
          tunnel: [w1965 errorcluster {"status"=TRUE, "code"=0, "source"="Init"} ("error out")] -> w1954
          tunnel: w1957 -> [w1965 _]
          frame False {
          }
          frame True {
          }
        }
        n1627 = case shown="Error" w1954 {
          selector: w1954 -> [w1975 w1993]
          tunnel: [w1978 w1997] -> w1964
          tunnel: [w1977 w1991] -> w1963
          tunnel: w1955 -> [w1976 w1995]
          frame No Error {
            n1628 = property class="Instr"(reference=w1976, error in=w1975) -> (reference out=w1973:refnum<visa-resource-name>, error out=w1974:errorcluster, "Serial Settings:Number of Bytes at Serial Port"=w1970:u32)
            n1629 = Greater?(x=w1970, y=u32 5) -> (0:w1969:bool)
            n1630 = Not(x=w1969) -> (.not. x?=→"Port 1a":bool)
            n1631 = while {
              tunnel: [w1986] -> w1977
              tunnel: [w1985] -> w1978
              tunnel: w1974 -> [w1984]
              tunnel: w1973 -> [w1983]
              stop <- TRUE stop-if-true
              n1632 = property class="Instr" props=["Serial Settings:Number of Bytes at Serial Port"](reference=w1983, error in=w1984) -> (reference out=w1988:refnum<visa-resource-name>, error out=w1987:errorcluster)  [unwired: 1 out]
              n1633 = VISA Read(VISA resource name=w1988, byte count=u32 50, error in (no error)=w1987) -> (VISA resource name out=w1985:refnum<visa-resource-name>, read buffer=w1980:string, error out=w1986:errorcluster)  [unwired: 1 out]
              n1634 = Wait (ms)(milliseconds to wait=u32 5) -> ()  [unwired: 1 out]
            }
          }
          frame Error {
            w2003 = u16 0 items=["None", "XON/XOFF", "RTS/CTS", "XON/XOFF & RTS/CTS", "DTR/DSR", "XON/XOFF & DTR/DSR"] ("flow control (0:none)  2")
            w2001 = u16 10 items=["1.0"=10, "1.5"=15, "2.0"=20] ("stop bits 2")
            w1999 = u16 0 items=["None", "Odd", "Even", "Mark", "Space"] ("parity 2")
            w2000 = u32 10000  # timeout (10sec)
            n1635 = VISA Close(VISA resource name=w1995, error in (no error)=w1993) -> (error out=w1996:errorcluster)
            n1636 = local write "Port 1a"(FALSE ("Port 1a")) -> ()
            n1637 = local read "Com Port 1"() -> (w1990:refnum<visa-resource-name>)
            n1638 = call <vilib>:"Clear Errors.vi"("error in (no error)"=w1996) -> ("error out"=w1994:errorcluster)  [unwired: 5 in, 1 out]
            n1639 = call-poly "VISA Configure Serial Port"("VISA resource name"=w1990, "timeout (10sec)"=w2000, "baud rate (9600)"=u32 250000 ("baud rate  2"), "data bits (8)"=u16 8 ("data bits  2"), "parity (0:none)"=w1999, "error in (no error)"=w1994, "stop bits (10: 1 bit)"=w2001, "flow control (0:none)"=w2003) -> ("VISA resource name out"=w2004:refnum<visa-resource-name>, "error out"=w2005:errorcluster)  [unwired: 6 in]
            n1640 = flat-sequence {
              tunnel: w2004 -> [w2007]
              tunnel: w2005 -> [w2006]
              tunnel: [w2007] -> w1997
              tunnel: [w2006] -> w1991
              frame #0 {
                n1641 = Wait (ms)(milliseconds to wait=u32 50) -> ()  [unwired: 1 out]
              }
            }
            "Residual Uno" <- ""
          }
        }
        n1642 = local read "Quit"() -> (w1952:bool)
        "Error Uno" <- w1957
      }
      n1643 = VISA Close(VISA resource name=w1950, error in (no error)=w1949) -> (error out=w1947:errorcluster)
      n1644 = call <vilib>:"Clear Errors.vi"("error in (no error)"=w1947) -> ()  [unwired: 5 in, 2 out]
    }
    frame Enabled {
    }
  }
  n1645 = while {
    stop <- w2018 stop-if-true
    # "V0OLTAGE TO STROKE (peice vise calibration)"
    n1646 = local read "LVDT MIN"() -> (w2010:dbl)
    n1647 = local read "LVDT Peak"() -> (w2009:dbl)
    n1648 = Wait (ms)(milliseconds to wait=u32 10) -> ()  [unwired: 1 out]
    n1649 = formula code="// Dynamic Parameterized Linear Interpolation Node\n// Inputs: vpp_val, voltages (Array), distances (Array)\n// Outputs: stroke\n\nint i = 0;\nint segments = 11; // 12 points make 11 interpolation segments\n\n// 1. Lower Boundary Clamp\nif (vpp_val <= voltages[0]) {\n    stroke = distances[0];\n}\n// 2. Upper Boundary Clamp\nelse if (vpp_val >= voltages[segments]) {\n    stroke = distances[segments];\n}\n// 3. Dynamic Segment Search Loop\nelse {\n    stroke = distances[0]; // Fallback baseline\n    for (i = 0; i < segments; i++) {\n        if (vpp_val >= voltages[i] && vpp_val <= voltages[i+1]) {\n            // Standard linear interpolation formula using array lookups\n            stroke = distances[i] + (vpp_val - voltages[i]) * (distances[i+1] - distances[i]) / (voltages[i+1] - voltages[i]);\n            break; // Segment found, safely exit the loop\n        }\n    }\n}"("vpp_val"=w2009, "voltages"="calibration values", "distances"="STROKE") -> ("stroke"=→"LVDT STROKE":dbl)
    n1650 = local read "Calibration Tare Value"() -> (w2014:dbl)
    n1651 = local read "Calibration Tare"() -> (w2012:bool)
    n1652 = Subtract(x=w2010, y=w2014) -> (x-y=→"LVDT STROKE  Calibration":dbl)
    n1653 = case shown="True" w2012 {
      selector: w2012 -> [_ w2020]
      tunnel: w2010 -> [_ w2021]
      frame False {
      }
      frame True {
        n1654 = Not(x=w2020) -> (.not. x?=w2019:bool)
        n1655 = local write "Calibration Tare"(w2019) -> ()
        "Calibration Tare Value" <- w2021
      }
    }
    n1656 = local read "Quit"() -> (w2018:bool)
  }
  n1657 = while {
    stop <- w2044 stop-if-true
    n1658 = local read "Due read"() -> (w2042:string)
    n1659 = call <vilib>:"High Resolution Polling Wait.vi"("seconds to wait"=0.02) -> ()  [unwired: 10 in, 1 out]
    n1660 = local read "Frictioin Force Raw"() -> (w2024:dbl)
    n1661 = Spreadsheet String To Array(delimiter (Tab)=";", format string="", spreadsheet string=w2042, array type (2D Dbl)=string[] []) -> (array=w2039:string[])
    n1662 = Fract/Exp String To Number(string=w2039) -> (number=w2038:dbl[])  [unwired: 3 in, 1 out]
    n1663 = call <vilib>:"Median Filter PtByPt.vi"("rank"=2, "x"=w2024) -> ("Filtered x"=→"Friction":dbl)  [unwired: 2 in, 1 out]
    n1664 = Index Array(array=w2038) -> (element #1=→"Sample Temperature":dbl, element #2=→"Target Sample Temperature":dbl, element #3=→"Current Duty Cycle":dbl, element #4=→"Ambient Temperature":dbl, element #5=→"Dac Status":dbl, element #6=→"Vpp":dbl, element #7=→"Active Error Code":dbl, element #8=→"Kp":dbl, element #9=→"Ki":dbl, element #10=→"Kd":dbl, element #11=→"SampleRaw":dbl, element #12=→"AmbRaw":dbl)  [unwired: 12 in]
    n1665 = local read "Quit"() -> (w2044:bool)
  }
  n1666 = while {
    shift-right: [w2058] -> w41
    shift-left: _ -> [w2050]
    shift-right: [w2045] -> w40
    shift-left: errorcluster {"status"=FALSE, "code"=0, "source"="Init"} ("error out") -> [w2052]
    tunnel: [w2047] -> w44
    tunnel: [w2057] -> _
    i -> [w2057]
    stop <- w2047 stop-if-true
    n1667 = local read "Com Port 2"() -> (w2051:refnum<visa-resource-name>)
    n1668 = local read "Port 2a"() -> (w2053:bool)
    n1669 = Unbundle(w2052) -> ("status"=→"Port 4":bool)  [unwired: 2 out]
    n1670 = call <vilib>:"High Resolution Polling Wait.vi"("seconds to wait"=0.02) -> ()  [unwired: 10 in, 1 out]
    n1671 = local read "Port 4"() -> (w2054:bool)
    n1672 = Not Equal?(x=w2051, y=w2050) -> (x != y?=w2049:bool)
    n1673 = Or(x=w2054, y=w2053) -> (x .or. y?=w2056:bool)
    n1674 = case shown="False" w2056 {
      frame False {
        w2061 = TRUE ("Visible")
        n1675 = property on="Port 2a" class="Bool (strict)"("Visible"=w2061) -> ()  [unwired: 2 in, 2 out]
        n1676 = property on="Port 4" class="Bool (strict)"("Visible"=w2061) -> ()  [unwired: 2 in, 2 out]
      }
      frame True {
        w2062 = TRUE ("Visible")
        n1677 = property on="Port 2a" class="Bool (strict)"("Visible"=w2062) -> ()  [unwired: 2 in, 2 out]
        n1678 = property on="Port 4" class="Bool (strict)"("Visible"=w2062) -> ()  [unwired: 2 in, 2 out]
      }
    }
    n1679 = case shown="True" w2049 {
      tunnel: [w2059 errorcluster {"status"=TRUE, "code"=0, "source"="Init"} ("error out")] -> w2048
      tunnel: w2052 -> [w2059 _]
      frame False {
      }
      frame True {
      }
    }
    n1680 = case shown="No Error" w2048 {
      selector: w2048 -> [w2075 w2106]
      tunnel: [w2068 w2111] -> w2058
      tunnel: [w2076 w2104] -> w2045
      tunnel: w2050 -> [w2077 w2109]
      frame No Error {
        n1681 = property class="Instr" props=["Serial Settings:Number of Bytes at Serial Port"](reference=w2077, error in=w2075) -> (reference out=w2069:refnum<visa-resource-name>, error out=w2074:errorcluster)  [unwired: 1 out]
        n1682 = while {
          tunnel: [w2085] -> w2070
          tunnel: [w2084] -> w2071
          tunnel: w2074 -> [w2083]
          tunnel: w2069 -> [w2082]
          tunnel: [w2081] -> _
          i -> [w2081]
          stop <- TRUE stop-if-true
          n1683 = property class="Instr" props=["Serial Settings:Number of Bytes at Serial Port"](reference=w2082, error in=w2083) -> (reference out=w2087:refnum<visa-resource-name>, error out=w2086:errorcluster)  [unwired: 1 out]
          n1684 = VISA Read(VISA resource name=w2087, byte count=u32 1000, error in (no error)=w2086) -> (VISA resource name out=w2084:refnum<visa-resource-name>, read buffer=→"Due read":string, error out=w2085:errorcluster)  [unwired: 1 out]
        }
        n1685 = local read "Due Write"() -> (w2067:string)
        n1686 = call <vilib>:"Trim Whitespace.vi"("string"=w2067) -> ("trimmed string"=w2066:string)  [unwired: 1 in]
        n1687 = Not Equal?(x=w2066, y="") -> (x != y?=w2072:bool)
        n1688 = VISA Flush I/O Buffer(VISA resource name=w2071) -> (VISA resource name out=w2064:refnum<visa-resource-name>, error out=→"error out 10":errorcluster)  [unwired: 2 in]
        n1689 = case shown="True" w2072 {
          tunnel: w2064 -> [w2089 w2094]
          tunnel: [w2089 w2098] -> w2068
          tunnel: w2070 -> [w2088 w2093]
          tunnel: [w2088 w2096] -> w2076
          tunnel: w2066 -> [_ w2092]
          tunnel: [_ w2095] -> _
          frame False {
            # "DATA  WRITE LOOP"
          }
          frame True {
            n1690 = Concatenate Strings(w2092, "\r\n") -> (w2091:string)
            n1691 = VISA Write(VISA resource name=w2094, write buffer=w2091, error in (no error)=w2093) -> (VISA resource name out=w2098:refnum<visa-resource-name>, return count=w2095:u32, error out=w2097:errorcluster)
            n1692 = flat-sequence {
              tunnel: w2097 -> [w2100]
              tunnel: [w2100] -> w2096
              frame #0 {
                n1693 = local write "Due Write"("" ("Command")) -> ()
                n1694 = Wait (ms)(milliseconds to wait=u32 5) -> ()  [unwired: 1 out]
              }
            }
          }
        }
        "Port 2a" <- TRUE ("Port 2a")
      }
      frame Error {
        w2117 = u16 0 items=["None", "XON/XOFF", "RTS/CTS", "XON/XOFF & RTS/CTS", "DTR/DSR", "XON/XOFF & DTR/DSR"] ("flow control (0:none)  2")
        w2115 = u16 10 items=["1.0"=10, "1.5"=15, "2.0"=20] ("stop bits 2")
        w2113 = u16 0 items=["None", "Odd", "Even", "Mark", "Space"] ("parity 2")
        w2114 = u32 10000  # timeout (10sec)
        n1695 = VISA Clear(VISA resource name=w2109, error in (no error)=w2106) -> (VISA resource name out=w2108:refnum<visa-resource-name>, error out=w2107:errorcluster)
        n1696 = VISA Close(VISA resource name=w2108, error in (no error)=w2107) -> (error out=w2110:errorcluster)